vi "Dresden R2R Sputter 03.02.2018 IY24.vi"() -> ()   [LabVIEW 2009] (continued)
                                frame #0 {
                                }
                                frame #1 {
                                n15348 = local write "Semi"(TRUE ("Semi")) -> ()
                                n15349 = local write "Error Message"("Start up process  cancelled\nbecause  CH1-VBV not closed.\nPlease check  CH1-VBV connections." ("Error Message")) -> ()
                                }
                                }
                                n15350 = local read "Ch1_Ch_vbv_di"() -> (w27355:bool)
                                n15351 = case shown="True" w27355 {
                                tunnel: [TRUE FALSE] -> w27354
                                frame #0 {
                                }
                                frame #1 {
                                n15352 = Wait Until Next ms Multiple(millisecond multiple=u32 200) -> ()  [unwired: 1 out]
                                n15353 = local write "Ch1_Ch_vbv_do"(FALSE ("Ch1_Tp_bv_do")) -> ()
                                }
                                }
                                n15354 = local read "Semi"() -> (w27353:bool)
                                n15355 = Or(x=w27354, y=w27353) -> (x .or. y?=w27352:bool)
                                }
                                }
                                frame #1 {
                                }
                                }
                                }
                                frame #1 {
                                n15356 = local read "Semi"() -> (w27365:bool)
                                n15357 = case shown="False" w27365 {
                                frame #0 {
                                n15358 = local write "Ch1_PV6"(TRUE ("P03")) -> ()
                                n15359 = Wait Until Next ms Multiple(millisecond multiple=u32 1000) -> ()  [unwired: 1 out]
                                }
                                frame #1 {
                                }
                                }
                                }
                                }
                              }
                              frame #1 {
                              }
                            }
                          }
                          frame #1 {
                            # "Close PL-VBV"
                            n15360 = local read "Semi"() -> (w27368:bool)
                            n15361 = case shown="False" w27368 {
                              frame #0 {
                                n15362 = stacked-sequence {
                                frame #0 {
                                n15363 = local read "Semi"() -> (w27369:bool)
                                n15364 = case shown="False" w27369 {
                                frame #0 {
                                n15365 = while {
                                i -> [w27376]
                                stop <- w27370 stop-if-true
                                n15366 = Greater?(x=w27376, y=50) -> (0:w27374:bool)
                                n15367 = case shown="True" w27374 {
                                frame #0 {
                                }
                                frame #1 {
                                n15368 = local write "Semi"(TRUE ("Semi")) -> ()
                                n15369 = local write "Error Message"("Start up process  cancelled\nbecause  PL1-VBV not closed.\nPlease check PL1-VBV connections." ("Error Message")) -> ()
                                }
                                }
                                n15370 = local read "Ch1_Pl_vbv_di"() -> (w27373:bool)
                                n15371 = case shown="True" w27373 {
                                tunnel: [TRUE FALSE] -> w27372
                                frame #0 {
                                }
                                frame #1 {
                                n15372 = Wait Until Next ms Multiple(millisecond multiple=u32 200) -> ()  [unwired: 1 out]
                                n15373 = local write "Ch1_Pl_vbv_do"(FALSE ("Ch1_Tp_bv_do")) -> ()
                                }
                                }
                                n15374 = local read "Semi"() -> (w27371:bool)
                                n15375 = Or(x=w27372, y=w27371) -> (x .or. y?=w27370:bool)
                                }
                                }
                                frame #1 {
                                }
                                }
                                }
                                frame #1 {
                                n15376 = local read "Semi"() -> (w27383:bool)
                                n15377 = case shown="False" w27383 {
                                frame #0 {
                                n15378 = local write "Ch1_PV7"(TRUE ("P03")) -> ()
                                n15379 = Wait Until Next ms Multiple(millisecond multiple=u32 1000) -> ()  [unwired: 1 out]
                                }
                                frame #1 {
                                }
                                }
                                }
                                }
                              }
                              frame #1 {
                              }
                            }
                          }
                          frame #2 {
                            # "Close CH1-ATM"
                            n15380 = local read "Semi"() -> (w27386:bool)
                            n15381 = case shown="False" w27386 {
                              frame #0 {
                                n15382 = stacked-sequence {
                                frame #0 {
                                n15383 = local read "Semi"() -> (w27387:bool)
                                n15384 = case shown="False" w27387 {
                                frame #0 {
                                n15385 = while {
                                i -> [w27394]
                                stop <- w27388 stop-if-true
                                n15386 = Greater?(x=w27394, y=50) -> (0:w27392:bool)
                                n15387 = case shown="True" w27392 {
                                frame #0 {
                                }
                                frame #1 {
                                n15388 = local write "Semi"(TRUE ("Semi")) -> ()
                                n15389 = local write "Error Message"("Start up process  cancelled\nbecause CH1-ATM not closed.\nPlease check CH1-ATM connections." ("Error Message")) -> ()
                                }
                                }
                                n15390 = local read "Ch1_Ch_atm_di"() -> (w27391:bool)
                                n15391 = case shown="True" w27391 {
                                tunnel: [TRUE FALSE] -> w27390
                                frame #0 {
                                }
                                frame #1 {
                                n15392 = Wait Until Next ms Multiple(millisecond multiple=u32 200) -> ()  [unwired: 1 out]
                                n15393 = local write "Ch1_Ch_atm_do"(TRUE ("Ch1_Tp_bv_do")) -> ()
                                }
                                }
                                n15394 = local read "Semi"() -> (w27389:bool)
                                n15395 = Or(x=w27390, y=w27389) -> (x .or. y?=w27388:bool)
                                }
                                }
                                frame #1 {
                                }
                                }
                                }
                                frame #1 {
                                n15396 = local read "Semi"() -> (w27401:bool)
                                n15397 = case shown="False" w27401 {
                                frame #0 {
                                n15398 = Wait Until Next ms Multiple(millisecond multiple=u32 1000) -> ()  [unwired: 1 out]
                                n15399 = local write "Ch1_PV8"(TRUE ("P03")) -> ()
                                }
                                frame #1 {
                                }
                                }
                                }
                                }
                              }
                              frame #1 {
                              }
                            }
                          }
                          frame #3 {
                            # "Close PL1-ATM"
                            n15400 = local read "Semi"() -> (w27404:bool)
                            n15401 = case shown="False" w27404 {
                              frame #0 {
                                n15402 = stacked-sequence {
                                frame #0 {
                                n15403 = local read "Semi"() -> (w27405:bool)
                                n15404 = case shown="False" w27405 {
                                frame #0 {
                                n15405 = while {
                                i -> [w27412]
                                stop <- w27406 stop-if-true
                                n15406 = Greater?(x=w27412, y=50) -> (0:w27410:bool)
                                n15407 = case shown="True" w27410 {
                                frame #0 {
                                }
                                frame #1 {
                                n15408 = local write "Semi"(TRUE ("Semi")) -> ()
                                n15409 = local write "Error Message"("Start up process  cancelled\nbecause PL1-ATM not closed.\nPlease check PL1-ATM connections." ("Error Message")) -> ()
                                }
                                }
                                n15410 = local read "Ch1_Pl_atm_di"() -> (w27409:bool)
                                n15411 = case shown="True" w27409 {
                                tunnel: [TRUE FALSE] -> w27408
                                frame #0 {
                                }
                                frame #1 {
                                n15412 = Wait Until Next ms Multiple(millisecond multiple=u32 200) -> ()  [unwired: 1 out]
                                n15413 = local write "Ch1_Pl_atm_do"(TRUE ("Ch1_Tp_bv_do")) -> ()
                                }
                                }
                                n15414 = local read "Semi"() -> (w27407:bool)
                                n15415 = Or(x=w27408, y=w27407) -> (x .or. y?=w27406:bool)
                                }
                                }
                                frame #1 {
                                }
                                }
                                }
                                frame #1 {
                                n15416 = local read "Semi"() -> (w27419:bool)
                                n15417 = case shown="False" w27419 {
                                frame #0 {
                                n15418 = local write "Ch1_PV9"(TRUE ("P03")) -> ()
                                n15419 = Wait Until Next ms Multiple(millisecond multiple=u32 1000) -> ()  [unwired: 1 out]
                                }
                                frame #1 {
                                }
                                }
                                }
                                }
                              }
                              frame #1 {
                              }
                            }
                          }
                          frame #4 {
                            # "START MP"
                            n15420 = local read "Semi"() -> (w27422:bool)
                            n15421 = case shown="False" w27422 {
                              frame #0 {
                                n15422 = stacked-sequence {
                                frame #0 {
                                n15423 = local read "Semi"() -> (w27423:bool)
                                n15424 = case shown="False" w27423 {
                                frame #0 {
                                n15425 = while {
                                i -> [w27430]
                                stop <- w27424 stop-if-true
                                n15426 = Greater?(x=w27430, y=50) -> (0:w27428:bool)
                                n15427 = case shown="True" w27428 {
                                frame #0 {
                                }
                                frame #1 {
                                n15428 = local write "Semi"(TRUE ("Semi")) -> ()
                                n15429 = local write "Error Message"("Start up process  cancelled\nbecause MP1 not started.\nPlease check MP1 connections." ("Error Message")) -> ()
                                }
                                }
                                n15430 = local read "Ch1_Mp_di"() -> (w27427:bool)
                                n15431 = case shown="False" w27427 {
                                tunnel: [FALSE TRUE] -> w27426
                                frame #0 {
                                n15432 = Wait Until Next ms Multiple(millisecond multiple=u32 200) -> ()  [unwired: 1 out]
                                n15433 = local write "Ch1_Mp_do"(TRUE ("Ch1_Tp_bv_do")) -> ()
                                }
                                frame #1 {
                                }
                                }
                                n15434 = local read "Semi"() -> (w27425:bool)
                                n15435 = Or(x=w27426, y=w27425) -> (x .or. y?=w27424:bool)
                                }
                                }
                                frame #1 {
                                }
                                }
                                }
                                frame #1 {
                                n15436 = local read "Semi"() -> (w27437:bool)
                                n15437 = case shown="False" w27437 {
                                frame #0 {
                                n15438 = local write "Ch1_PV10"(TRUE ("P03")) -> ()
                                n15439 = Wait Until Next ms Multiple(millisecond multiple=u32 1000) -> ()  [unwired: 1 out]
                                }
                                frame #1 {
                                }
                                }
                                }
                                }
                              }
                              frame #1 {
                              }
                            }
                          }
                          frame #5 {
                            # "CHECK PL-PRESSURE"
                            n15440 = local read "Semi"() -> (w27440:bool)
                            n15441 = case shown="False" w27440 {
                              frame #0 {
                                n15442 = stacked-sequence {
                                frame #0 {
                                n15443 = local read "Semi"() -> (w27441:bool)
                                n15444 = case shown="False" w27441 {
                                frame #0 {
                                n15445 = while {
                                i -> [w27450]
                                stop <- w27445 stop-if-true
                                n15446 = Greater?(x=w27450, y=240) -> (0:w27448:bool)
                                n15447 = case shown="True" w27448 {
                                frame #0 {
                                }
                                frame #1 {
                                n15448 = local write "Semi"(TRUE ("Semi")) -> ()
                                n15449 = local write "Error Message"("Start up process was cancelled.\nPlease check Pipeline \nvacuum connections." ("Error Message")) -> ()
                                }
                                }
                                n15450 = local read "Pl_pg_press_ch1"() -> (w27444:dbl)
                                n15451 = Less?(x=w27444, y=0.9) -> (x < y?=w27442:bool)
                                n15452 = case shown="False" w27442 {
                                tunnel: [FALSE TRUE] -> w27447
                                frame #0 {
                                n15453 = Wait Until Next ms Multiple(millisecond multiple=u32 200) -> ()  [unwired: 1 out]
                                }
                                frame #1 {
                                }
                                }
                                n15454 = local read "Semi"() -> (w27446:bool)
                                n15455 = Or(x=w27447, y=w27446) -> (x .or. y?=w27445:bool)
                                }
                                }
                                frame #1 {
                                }
                                }
                                }
                                frame #1 {
                                n15456 = local read "Semi"() -> (w27456:bool)
                                n15457 = case shown="False" w27456 {
                                frame #0 {
                                n15458 = local write "Ch1_PV11"(TRUE ("P03")) -> ()
                                n15459 = Wait Until Next ms Multiple(millisecond multiple=u32 1000) -> ()  [unwired: 1 out]
                                }
                                frame #1 {
                                }
                                }
                                }
                                }
                              }
                              frame #1 {
                              }
                            }
                          }
                          frame #6 {
                            # "CHECK CH-PRESSURE"
                            n15460 = local read "Semi"() -> (w27459:bool)
                            n15461 = case shown="False" w27459 {
                              frame #0 {
                                n15462 = stacked-sequence {
                                frame #0 {
                                n15463 = local read "Semi"() -> (w27460:bool)
                                n15464 = case shown="False" w27460 {
                                frame #0 {
                                n15465 = while {
                                i -> [w27469]
                                stop <- w27464 stop-if-true
                                n15466 = Greater?(x=w27469, y=50) -> (0:w27467:bool)
                                n15467 = case shown="True" w27467 {
                                frame #0 {
                                }
                                frame #1 {
                                n15468 = local write "Semi"(TRUE ("Semi")) -> ()
                                n15469 = local write "Error Message"("Start up process was cancelled.\nPlease check chamber \nvacuum connections." ("Error Message")) -> ()
                                }
                                }
                                n15470 = local read "Ch1_pressure"() -> (w27463:dbl)
                                n15471 = Less?(x=w27463, y=0.9) -> (x < y?=w27461:bool)
                                n15472 = case shown="False" w27461 {
                                tunnel: [FALSE TRUE] -> w27466
                                frame #0 {
                                n15473 = Wait Until Next ms Multiple(millisecond multiple=u32 200) -> ()  [unwired: 1 out]
                                }
                                frame #1 {
                                }
                                }
                                n15474 = local read "Semi"() -> (w27465:bool)
                                n15475 = Or(x=w27466, y=w27465) -> (x .or. y?=w27464:bool)
                                }
                                }
                                frame #1 {
                                }
                                }
                                }
                                frame #1 {
                                n15476 = local read "Semi"() -> (w27475:bool)
                                n15477 = case shown="False" w27475 {
                                frame #0 {
                                n15478 = Wait Until Next ms Multiple(millisecond multiple=u32 1000) -> ()  [unwired: 1 out]
                                n15479 = local write "Ch1_PV12"(TRUE ("P03")) -> ()
                                }
                                frame #1 {
                                }
                                }
                                }
                                }
                              }
                              frame #1 {
                              }
                            }
                          }
                          frame #7 {
                            # "OPEN TP-BV"
                            n15480 = local read "Semi"() -> (w27478:bool)
                            n15481 = case shown="False" w27478 {
                              frame #0 {
                                n15482 = stacked-sequence {
                                frame #0 {
                                n15483 = local read "Semi"() -> (w27479:bool)
                                n15484 = case shown="False" w27479 {
                                frame #0 {
                                n15485 = while {
                                i -> [w27486]
                                stop <- w27481 stop-if-true
                                n15486 = Greater?(x=w27486, y=50) -> (0:w27484:bool)
                                n15487 = case shown="True" w27484 {
                                frame #0 {
                                }
                                frame #1 {
                                n15488 = local write "Semi"(TRUE ("Semi")) -> ()
                                n15489 = local write "Error Message"("Start up process  cancelled\nbecause  TP-BV not opened.\nPlease check TP-BV1 connections." ("Error Message")) -> ()
                                }
                                }
                                n15490 = local read "Ch1_Tp_bv_di"() -> (w27480:bool)
                                n15491 = case shown="False" w27480 {
                                tunnel: [FALSE TRUE] -> w27483
                                frame #0 {
                                n15492 = Wait Until Next ms Multiple(millisecond multiple=u32 200) -> ()  [unwired: 1 out]
                                n15493 = local write "Ch1_Tp_bv_do"(TRUE ("Ch1_Tp_bv_do")) -> ()
                                }
                                frame #1 {
                                }
                                }
                                n15494 = local read "Semi"() -> (w27482:bool)
                                n15495 = Or(x=w27483, y=w27482) -> (x .or. y?=w27481:bool)
                                }
                                }
                                frame #1 {
                                }
                                }
                                }
                                frame #1 {
                                n15496 = local read "Semi"() -> (w27493:bool)
                                n15497 = case shown="False" w27493 {
                                frame #0 {
                                n15498 = local write "Ch1_PV13"(TRUE ("P03")) -> ()
                                n15499 = Wait Until Next ms Multiple(millisecond multiple=u32 1000) -> ()  [unwired: 1 out]
                                }
                                frame #1 {
                                }
                                }
                                }
                                }
                              }
                              frame #1 {
                              }
                            }
                          }
                          frame #8 {
                            # "OPEN PC-BV"
                            n15500 = local read "Semi"() -> (w27496)
                            n15501 = case shown="False" w27496 {
                              frame #0 {
                                n15502 = stacked-sequence {
                                frame #0 {
                                n15503 = local read "Semi"() -> (w27497)
                                n15504 = case shown="False" w27497 {
                                frame #0 {
                                n15505 = stacked-sequence {
                                frame #0 {
                                n15506 = local read "Semi"() -> (w27498:bool)
                                n15507 = case shown="False" w27498 {
                                frame #0 {
                                n15508 = local write "Pc_bv1_auto_open"(TRUE ("Tp1_auto_start")) -> ()
                                }
                                frame #1 {
                                }
                                }
                                }
                                frame #1 {
                                n15509 = local read "Semi"() -> (w27500:bool)
                                n15510 = case shown="False" w27500 {
                                frame #0 {
                                n15511 = Wait (ms)(milliseconds to wait=u32 1000) -> ()  [unwired: 1 out]
                                }
                                frame #1 {
                                }
                                }
                                }
                                frame #2 {
                                n15512 = local read "Semi"() -> (w27502:bool)
                                n15513 = case shown="False" w27502 {
                                frame #0 {
                                n15514 = while {
                                i -> [w27508]
                                stop <- w27504 stop-if-true
                                n15515 = local read "Pc_bv_opened_ch1"() -> (w27506:bool)
                                n15516 = Greater?(x=w27508, y=120) -> (0:w27507:bool)
                                n15517 = local read "Semi"() -> (w27505:bool)
                                n15518 = Compound Arithmetic op=OR(w27505, w27506, w27507) -> (w27504:bool)
                                n15519 = Wait (ms)(milliseconds to wait=u32 500) -> ()  [unwired: 1 out]
                                }
                                }
                                frame #1 {
                                }
                                }
                                }
                                frame #3 {
                                n15520 = local read "Semi"() -> (w27510:bool)
                                n15521 = case shown="False" w27510 {
                                frame #0 {
                                n15522 = local read "Pc_bv_opened_ch1"() -> (w27511:bool)
                                n15523 = case shown="False" w27511 {
                                frame #0 {
                                n15524 = local write "Pc_bv1_auto_open"(TRUE ("Pc_bv1_auto_open")) -> ()
                                }
                                frame #1 {
                                }
                                }
                                }
                                frame #1 {
                                }
                                }
                                }
                                frame #4 {
                                n15525 = local read "Semi"() -> (w27513:bool)
                                n15526 = case shown="False" w27513 {
                                frame #0 {
                                n15527 = local read "Pc_bv_opened_ch1"() -> (w27514:bool)
                                n15528 = case shown="False" w27514 {
                                frame #0 {
                                n15529 = Wait (ms)(milliseconds to wait=u32 1000) -> ()  [unwired: 1 out]
                                }
                                frame #1 {
                                }
                                }
                                }
                                frame #1 {
                                }
                                }
                                }
                                frame #5 {
                                n15530 = local read "Semi"() -> (w27516:bool)
                                n15531 = case shown="False" w27516 {
                                frame #0 {
                                n15532 = while {
                                i -> [w27522]
                                stop <- w27518 stop-if-true
                                n15533 = local read "Pc_bv_opened_ch1"() -> (w27520:bool)
                                n15534 = Greater?(x=w27522, y=120) -> (0:w27521:bool)
                                n15535 = local read "Semi"() -> (w27519:bool)
                                n15536 = Compound Arithmetic op=OR(w27519, w27520, w27521) -> (w27518:bool)
                                n15537 = Wait (ms)(milliseconds to wait=u32 500) -> ()  [unwired: 1 out]
                                }
                                }
                                frame #1 {
                                }
                                }
                                }
                                frame #6 {
                                n15538 = local read "Semi"() -> (w27524)
                                n15539 = case shown="False" w27524 {
                                frame #0 {
                                n15540 = local read "Pc_bv_opened_ch1"() -> (w27525)
                                n15541 = case shown="False" w27525 {
                                frame #0 {
                                n15542 = local write "Error Message"("Start up process  cancelled\nbecause  PC-BV not opened.\nPlease check PC-BV1 connections." ("Error Message")) -> ()
                                n15543 = Wait (ms)(milliseconds to wait=i32? 1000) -> ()  [unwired: 1 out]
                                }
                                frame #1 {
                                }
                                }
                                }
                                frame #1 {
                                }
                                }
                                }
                                }
                                }
                                frame #1 {
                                }
                                }
                                }
                                frame #1 {
                                n15544 = local read "Semi"() -> (w27528)
                                n15545 = case shown="False" w27528 {
                                frame #0 {
                                n15546 = local write "Ch1_PV14"(T/1 ("P03")) -> ()
                                n15547 = Wait Until Next ms Multiple(millisecond multiple=i32? 1000) -> ()  [unwired: 1 out]
                                }
                                frame #1 {
                                }
                                }
                                }
                                }
                              }
                              frame #1 {
                              }
                            }
                          }
                          frame #9 {
                            # "OPEN/CLOSE TRNS GV-BP2"
                            n15548 = local read "Semi"() -> (w27531)
                            n15549 = case shown="False" w27531 {
                              frame #0 {
                                n15550 = stacked-sequence {
                                frame #0 {
                                n15551 = local read "Semi"() -> (w27532)
                                n15552 = case shown="False" w27532 {
                                frame #0 {
                                n15553 = while {
                                i -> [w27541]
                                stop <- w27536 stop-if-true
                                n15554 = Greater?(x=w27541, y=i32? 50) -> (0:w27539)
                                n15555 = case shown="True" w27539 {
                                frame #0 {
                                }
                                frame #1 {
                                n15556 = local read "Ch2_pressure"() -> (w27555)
                                n15557 = Less?(x=w27555, y=i32? 1) -> (x < y?=w27554)
                                n15558 = case shown="True" w27554 {
                                frame #0 {
                                n15559 = local write "Error Message"("Start up process  cancelled\nbecause  Trns GV-BP2 not closed.\nPlease check \nTrns GV-BP2 connections." ("Error Message")) -> ()
                                }
                                frame #1 {
                                n15560 = local write "Error Message"("Start up process  cancelled\nbecause  Trns GV-BP2 not opened.\nPlease check \nTrns GV-BP2 connections." ("Error Message")) -> ()
                                }
                                }
                                n15561 = local write "Semi"(T/1 ("Semi")) -> ()
                                }
                                }
                                n15562 = local read "Ch2_pressure"() -> (w27535)
                                n15563 = Less?(x=w27535, y=i32? 1) -> (x < y?=w27533)
                                n15564 = case shown="True" w27533 {
                                tunnel: [w27543 w27549] -> w27538
                                frame #0 {
                                n15565 = local read "Ch1_Trns_gv_bp2_di"() -> (w27542)
                                n15566 = case shown="True" w27542 {
                                tunnel: [T/1 i16? 0] -> w27543
                                frame #0 {
                                }
                                frame #1 {
                                n15567 = local write "Ch1_Trns_gv_bp2_do"(i16? 0 ("Ch1_Tp_bv_do")) -> ()
                                n15568 = Wait Until Next ms Multiple(millisecond multiple=i32? 200) -> ()  [unwired: 1 out]
                                }
                                }
                                }
                                frame #1 {
                                n15569 = local read "Ch1_Trns_gv_bp2_di"() -> (w27548)
                                n15570 = case shown="False" w27548 {
                                tunnel: [i16? 0 T/1] -> w27549
                                frame #0 {
                                n15571 = local write "Ch1_Trns_gv_bp2_do"(T/1 ("Ch1_Tp_bv_do")) -> ()
                                n15572 = Wait Until Next ms Multiple(millisecond multiple=i32? 200) -> ()  [unwired: 1 out]
                                }
                                frame #1 {
                                }
                                }
                                }
                                }
                                n15573 = local read "Semi"() -> (w27537)
                                n15574 = Or(x=w27538, y=w27537) -> (x .or. y?=w27536)
                                }
                                }
                                frame #1 {
                                }
                                }
                                }
                                frame #1 {
                                n15575 = local read "Semi"() -> (w27560)
                                n15576 = case shown="False" w27560 {
                                frame #0 {
                                n15577 = local write "Ch1_PV15"(T/1 ("P03")) -> ()
                                n15578 = Wait Until Next ms Multiple(millisecond multiple=i32? 1000) -> ()  [unwired: 1 out]
                                }
                                frame #1 {
                                }
                                }
                                }
                                }
                              }
                              frame #1 {
                              }
                            }
                          }
                          frame #10 {
                            # "CHECK CH-PRESSURE"
                            n15579 = local read "Semi"() -> (w27563)
                            n15580 = case shown="False" w27563 {
                              frame #0 {
                                n15581 = stacked-sequence {
                                frame #0 {
                                n15582 = local read "Semi"() -> (w27564)
                                n15583 = case shown="False" w27564 {
                                frame #0 {
                                n15584 = while {
                                i -> [w27573]
                                stop <- w27568 stop-if-true
                                n15585 = Greater?(x=w27573, y=i32? 600) -> (0:w27571)
                                n15586 = case shown="True" w27571 {
                                frame #0 {
                                }
                                frame #1 {
                                n15587 = local write "Semi"(T/1 ("Semi")) -> ()
                                n15588 = local write "Error Message"("Start up process was cancelled.\nPlease check chamber \nvacuum connections." ("Error Message")) -> ()
                                }
                                }
                                n15589 = local read "Ch1_pressure"() -> (w27567)
                                n15590 = Less?(x=w27567, y=dbl? 0.9) -> (x < y?=w27565)
                                n15591 = case shown="True" w27565 {
                                tunnel: [i16? 0 T/1] -> w27570
                                frame #0 {
                                n15592 = Wait Until Next ms Multiple(millisecond multiple=i32? 500) -> ()  [unwired: 1 out]
                                }
                                frame #1 {
                                }
                                }
                                n15593 = local read "Semi"() -> (w27569)
                                n15594 = Or(x=w27570, y=w27569) -> (x .or. y?=w27568)
                                }
                                }
                                frame #1 {
                                }
                                }
                                }
                                frame #1 {
                                n15595 = local read "Semi"() -> (w27579)
                                n15596 = case shown="False" w27579 {
                                frame #0 {
                                n15597 = local write "Ch1_PV16"(T/1 ("P03")) -> ()
                                n15598 = Wait Until Next ms Multiple(millisecond multiple=i32? 1000) -> ()  [unwired: 1 out]
                                }
                                frame #1 {
                                }
                                }
                                }
                                }
                              }
                              frame #1 {
                              }
                            }
                          }
                          frame #11 {
                            # "OPEN BG-BV"
                            n15599 = local read "Semi"() -> (w27582)
                            n15600 = case shown="False" w27582 {
                              frame #0 {
                                n15601 = stacked-sequence {
                                frame #0 {
                                n15602 = local read "Semi"() -> (w27583)
                                n15603 = case shown="False" w27583 {
                                frame #0 {
                                n15604 = while {
                                i -> [w27590]
                                stop <- w27585 stop-if-true
                                n15605 = Greater?(x=w27590, y=i32? 50) -> (0:w27588)
                                n15606 = case shown="True" w27588 {
                                frame #0 {
                                }
                                frame #1 {
                                n15607 = local write "Semi"(T/1 ("Semi")) -> ()
                                n15608 = local write "Error Message"("Start up process  cancelled\nbecause  BG-BV not opened.\nPlease check BG-BV1 connections." ("Error Message")) -> ()
                                }
                                }
                                n15609 = local read "Ch1_Bg_bv_di"() -> (w27584)
                                n15610 = case shown="False" w27584 {
                                tunnel: [i16? 0 T/1] -> w27587
                                frame #0 {
                                n15611 = Wait Until Next ms Multiple(millisecond multiple=i32? 200) -> ()  [unwired: 1 out]
                                n15612 = local write "Ch1_Bg_bv_do"(T/1 ("Ch1_Tp_bv_do")) -> ()
                                }
                                frame #1 {
                                }
                                }
                                n15613 = local read "Semi"() -> (w27586)
                                n15614 = Or(x=w27587, y=w27586) -> (x .or. y?=w27585)
                                }
                                }
                                frame #1 {
                                }
                                }
                                }
                                frame #1 {
                                n15615 = local read "Semi"() -> (w27597)
                                n15616 = case shown="False" w27597 {
                                frame #0 {
                                n15617 = local write "Ch1_PV17"(T/1 ("P03")) -> ()
                                n15618 = Wait Until Next ms Multiple(millisecond multiple=i32? 1000) -> ()  [unwired: 1 out]
                                }
                                frame #1 {
                                }
                                }
                                }
                                }
                              }
                              frame #1 {
                              }
                            }
                          }
                          frame #12 {
                            # "CHECK CH-PRESSURE"
                            n15619 = local read "Semi"() -> (w27600)
                            n15620 = case shown="False" w27600 {
                              frame #0 {
                                n15621 = stacked-sequence {
                                frame #0 {
                                n15622 = local read "Semi"() -> (w27601)
                                n15623 = case shown="False" w27601 {
                                frame #0 {
                                n15624 = while {
                                i -> [w27610]
                                stop <- w27605 stop-if-true
                                n15625 = Greater?(x=w27610, y=i32? 240) -> (0:w27608)
                                n15626 = case shown="True" w27608 {
                                frame #0 {
                                }
                                frame #1 {
                                n15627 = local write "Semi"(T/1 ("Semi")) -> ()
                                n15628 = local write "Error Message"("Start up process was cancelled.\nPlease check chamber \nvacuum connections." ("Error Message")) -> ()
                                }
                                }
                                n15629 = local read "Ch1_pressure"() -> (w27604)
                                n15630 = Less?(x=w27604, y=dbl? 0.9) -> (x < y?=w27602)
                                n15631 = case shown="False" w27602 {
                                tunnel: [i16? 0 T/1] -> w27607
                                frame #0 {
                                n15632 = Wait Until Next ms Multiple(millisecond multiple=i32? 500) -> ()  [unwired: 1 out]
                                }
                                frame #1 {
                                }
                                }
                                n15633 = local read "Semi"() -> (w27606)
                                n15634 = Or(x=w27607, y=w27606) -> (x .or. y?=w27605)
                                }
                                }
                                frame #1 {